vi "Visualizacion_NEW.vi"() -> ()   [LabVIEW 2021] (continued)
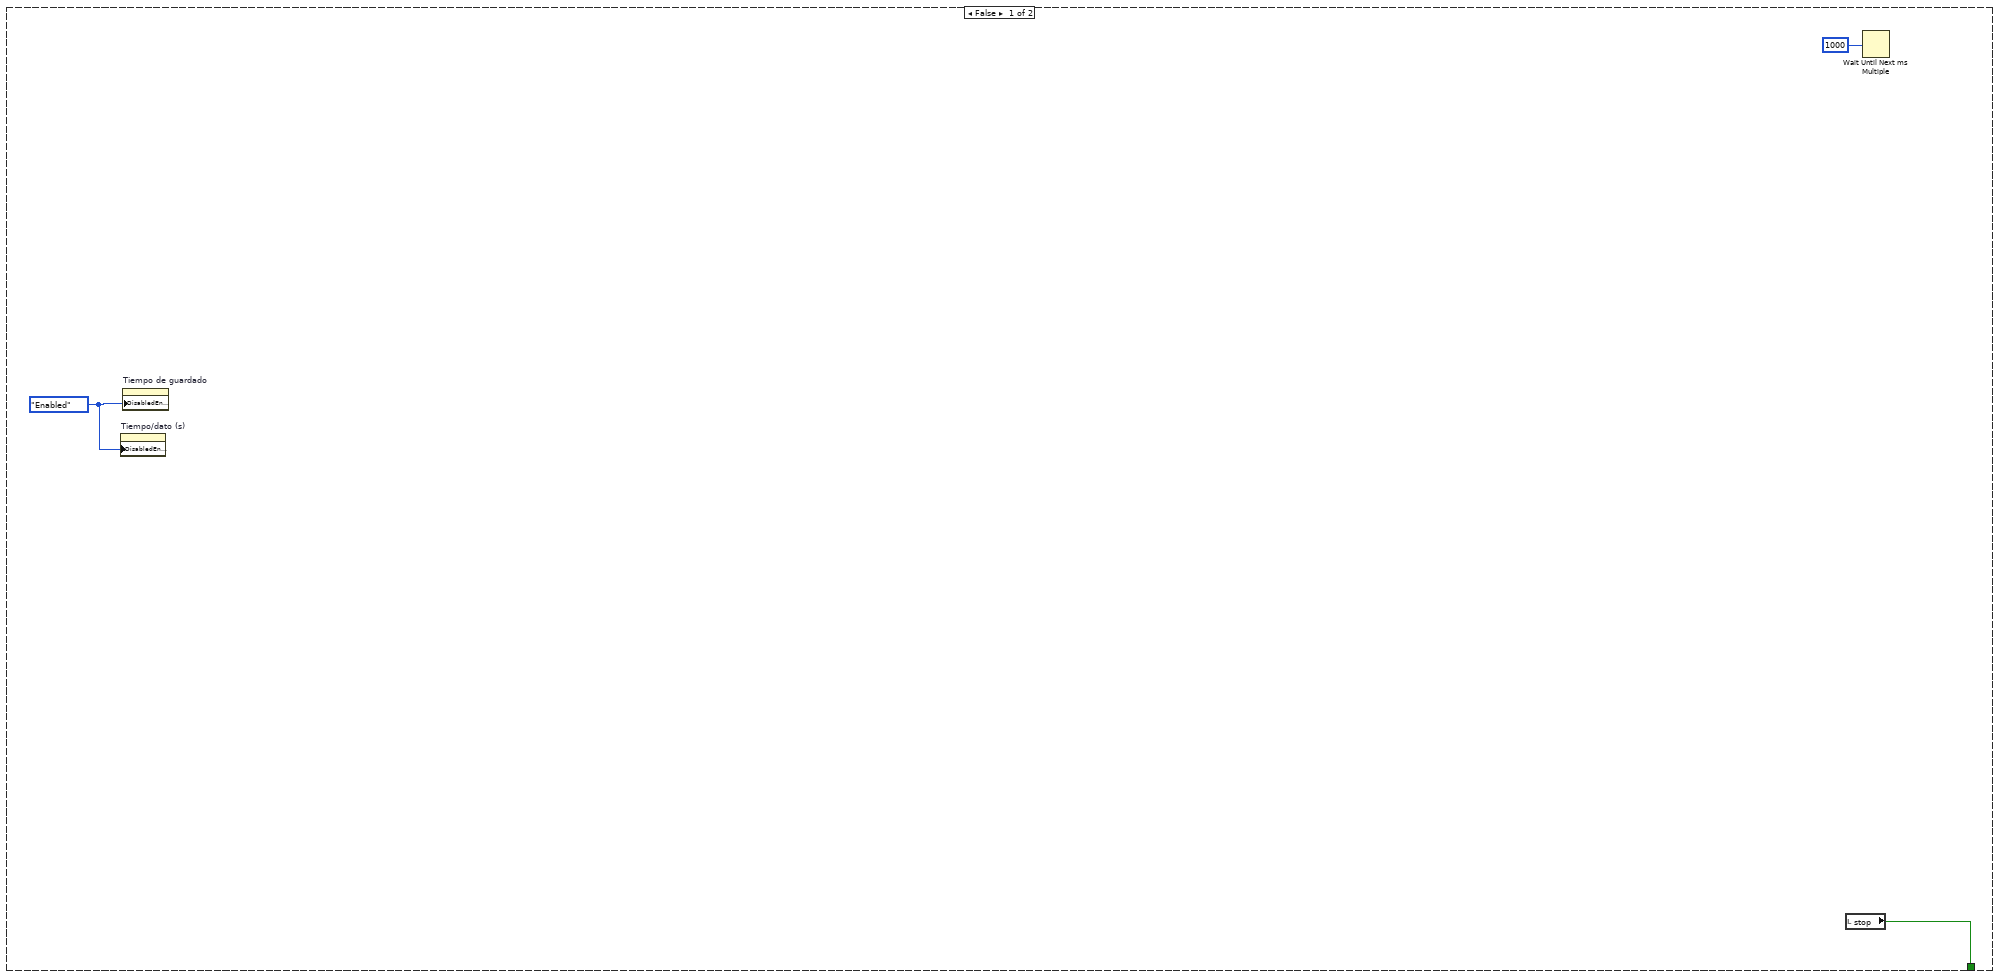
[diagram p2: hidden frame]
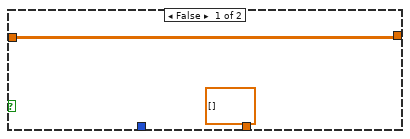
[diagram p3: hidden frame]
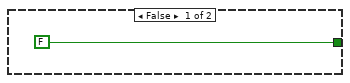
[diagram p4: hidden frame]
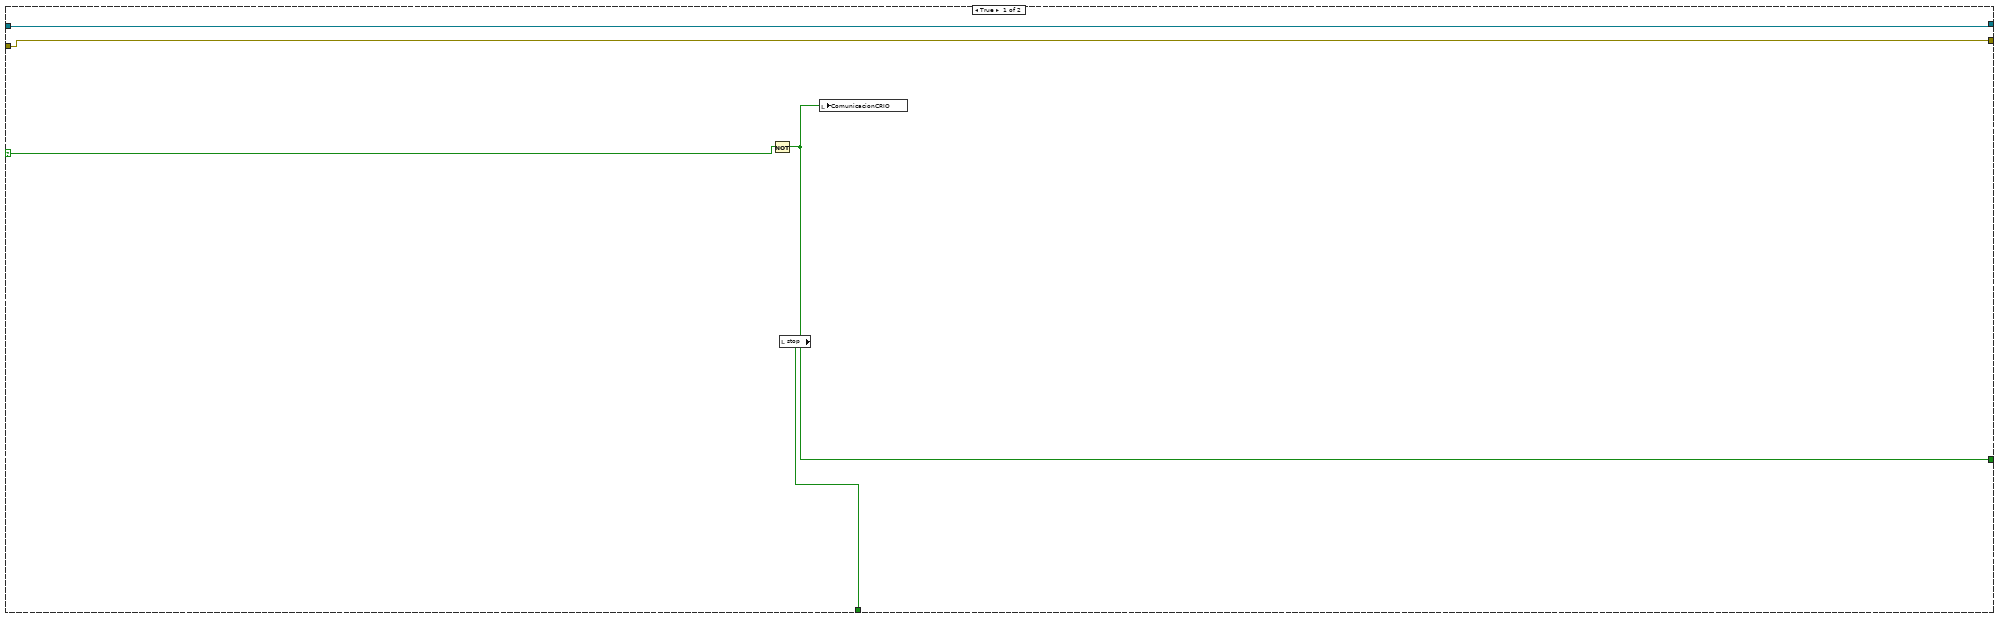
[diagram p6: hidden frame]
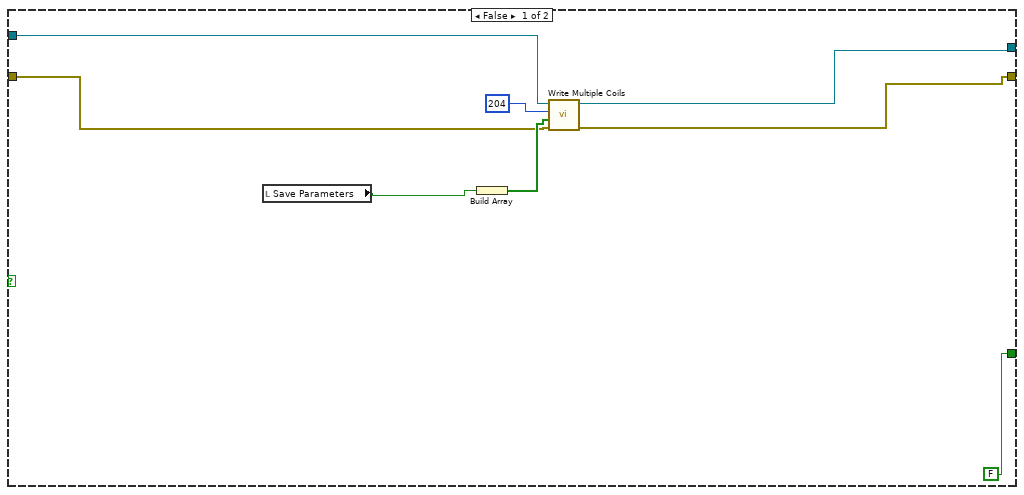
[diagram p8: hidden frame]
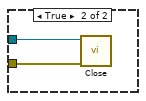
[diagram p9: hidden frame]
                frame False {
                }
                frame True {
                  n111 = flat-sequence {
                    tunnel: w160 -> [w172]
                    tunnel: w159 -> [w171]
                    tunnel: w158 -> [w170]
                    tunnel: w157 -> [w169]
                    tunnel: [w169] -> w155
                    tunnel: [w164] -> w152
                    tunnel: [w163] -> w150
                    tunnel: w155 -> [w185]
                    tunnel: [w185] -> w154
                    tunnel: [w184] -> w153
                    tunnel: w152 -> [w184]
                    tunnel: [w183] -> w151
                    tunnel: w150 -> [w183]
                    tunnel: [FALSE ("Warning saved")] -> w149
                    tunnel: [w189] -> w156
                    tunnel: w154 -> [w189]
                    tunnel: w153 -> [w188]
                    tunnel: w151 -> [w187]
                    tunnel: w149 -> [w186]
                    frame #0 {
                      n112 = disable-structure shown="Disabled" {
                        frame Disabled {
                          n113 = call <vilib>:"Application Directory.vi"() -> ("Application Directory"=w178:path)
                          n114 = Build Path(base path=w178) -> (appended path=w177:path)  [unwired: 1 in]
                          n115 = Build Path(base path=w177, name or relative path=path "data CC.tdms") -> ()  [unwired: 1 out]
                        }
                        frame Enabled {
                        }
                      }
                      n116 = TDMS Open(10:T6."open or create" ("operation (0:open)"), 11:w170) -> (0:w174:errorcluster, 3:w175:refnum<k34>)  [unwired: 5 in]
                      n117 = local read "W to save"() -> (w161:string[][])
                      n118 = TDMS Write(0:w175, 5:"Cámara climática" ("group name in (Untitled)"), 7:w172, 9:w171, 11:w174) -> (4:w168:refnum<k34>, 15:w167:errorcluster)  [unwired: 1 in, 2 out]
                      n119 = Transpose 2D Array(2D array=w161) -> (transposed array=w162:string[][])
                      n120 = TDMS Write(0:w168, 5:"Warnings y Errores" ("group name in (Untitled)"), 7:string[] ["Time", "id", "Description"] ("channel name(s) in (Untitled)"), 9:w162, 11:w167) -> (4:w163:refnum<k34>, 15:w164:errorcluster)  [unwired: 1 in, 2 out]
                    }
                    frame #1 {
                      n121 = local write "Warning saved"(TRUE ("Warning saved")) -> ()
                      n122 = Wait (ms)(milliseconds to wait=u32 300) -> ()  [unwired: 1 out]
                    }
                    frame #2 {
                      n123 = TDMS Close(8:w188, 11:w187) -> ()  [unwired: 2 out]
                      n124 = local write "Warning saved"(w186) -> ()
                    }
                  }
                }
              }
              n125 = Transpose 2D Array(2D array=w132) -> (transposed array=w131:dbl[][])
              n126 = Multiply(x="Tiempo/dato (s)", y=u32 1000) -> (x*y=w87:u32)
              n127 = Wait Until Next ms Multiple(millisecond multiple=w87) -> ()  [unwired: 1 out]
            }
          }
        }
      }
      n128 = while {
        tunnel: w18 -> [_]
        tunnel: w17 -> [_]
        tunnel: w16 -> [_]
        stop <- w190 stop-if-true
        n129 = flat-sequence {
          tunnel: [w199] -> w193
          tunnel: [w198] -> w192
          tunnel: [w197] -> w191
          tunnel: [w196] -> w190
          tunnel: w193 -> [w379]
          tunnel: w192 -> [w378]
          tunnel: w191 -> [w377]
          frame #0 {
            n130 = call-poly <vilib>:"Create Master Instance.vi"("address"="192.168.111.60") -> ("error out"=w195:errorcluster, "TCP master instance"=w200:refnum<class "Modbus Master.lvclass">)  [unwired: 9 in]
            "Comunicacion Modbus" <- w195
            n131 = Unbundle By Name(w195) -> ("status"=w194:bool)
            n132 = case shown="False" w194 {
              selector: w194 -> [w203 _]
              tunnel: w200 -> [w206 w212]
              tunnel: [w204 w211] -> w199
              tunnel: [w206 w210] -> w198
              tunnel: [w205 w209] -> w197
              tunnel: [w202 w208] -> w196
              tunnel: w195 -> [w205 w207]
              frame True {
                n133 = Not(x=w203) -> (.not. x?=w204:bool)
                n134 = local read "stop"() -> (w202:bool)
                n135 = local write "ComunicacionCRIO"(w204) -> ()
              }
              frame False {
                n136 = while {
                  shift-right: [w214] -> w210
                  shift-left: w212 -> [w282]
                  shift-right: [w213] -> w209
                  shift-left: w207 -> [w281]
                  tunnel: [w278] -> w211
                  tunnel: [w276] -> w208
                  stop <- w280 stop-if-true
                  n137 = call-dynamic "Read Coils.vi"("error in (no error)"=w281, "number of coils"=u16 23, "starting address"=u16 1, "Modbus master in"=w282) -> ("error out"=w267:errorcluster, "coil values"=w271:bool[], "Modbus master out"=w268:refnum<class "Modbus Master.lvclass">)  [unwired: 5 in]
                  n138 = local write "coil values"(w271) -> ()
                  n139 = call-dynamic "Read Coils.vi"("error in (no error)"=w267, "number of coils"=u16 1, "starting address"=u16 4, "Modbus master in"=w268) -> ("error out"=w265:errorcluster, "coil values"=w262:bool[], "Modbus master out"=w266:refnum<class "Modbus Master.lvclass">)  [unwired: 5 in]
                  n140 = Index Array(array=w262, index=0) -> (element=→"DO H2 Lab":bool)
                  n141 = call-dynamic "Read Holding Registers.vi"("error in (no error)"=w265, "number of holding registers"=u16 53, "starting address"=u16 100, "Modbus master in"=w266) -> ("error out"=w274:errorcluster, "register values"=w284:u16[], "Modbus master out"=w275:refnum<class "Modbus Master.lvclass">)  [unwired: 5 in]
                  n142 = Split 1D Array(array=w284, index=9) -> (first subarray=w283:u16[], second subarray=w288:u16[])
                  n143 = Array Size(array=w288) -> (size(s)=w287:i32)
                  n144 = Quotient & Remainder(x=w287, y=2) -> (floor(x/y)=w285:i32)  [unwired: 1 out]
                  n145 = for {
                    N: w285 -> [_]
                    tunnel: w288 -> [w369]
                    tunnel: [w366] -> w269 mode=indexing
                    i -> [w376]
                    n146 = Multiply(x=2, y=w376) -> (x*y=w374:i32)
                    n147 = Add(x=w374, y=1) -> (x+y=w372:i32)
                    n148 = Index Array(array=w369, index #1=w374, index #2=w372) -> (element #1=w371:u16, element #2=w370:u16)
                    n149 = Join Numbers(hi=w371, lo=w370) -> ((hi.lo)=w368:u32)
                    n150 = To Single Precision Float(number=w368) -> (single precision float=w365:sgl)
                    n151 = Subtract(x=w365, y=sgl 10000.0) -> (x-y=w363:sgl)
                    n152 = Divide(x=w363, y=sgl 100.0) -> (x/y=w366:sgl)
                  }
                  n153 = for {
                    tunnel: w283 -> [w362] mode=indexing
                    tunnel: [w360] -> w270 mode=indexing
                    n154 = Subtract(x=w362, y=u16 10000) -> (x-y=w360:u16)
                  }
                  n155 = local read "Coils write"() -> (w272:bool[])
                  n156 = local write "Int values"(w270) -> ()
                  n157 = local write "SGL values"(w269) -> ()
                  n158 = call-dynamic "Write Multiple Coils.vi"("error in (no error)"=w274, "coil values"=w272, "starting address"=u16 200, "Modbus master in"=w275) -> ("error out"=w255:errorcluster, "Modbus master out"=w256:refnum<class "Modbus Master.lvclass">)  [unwired: 6 in]
                  n159 = Build Array("Test PID (ºC)") -> (w253:bool[])
                  n160 = call-dynamic "Write Multiple Coils.vi"("error in (no error)"=w255, "coil values"=w253, "starting address"=u16 250, "Modbus master in"=w256) -> ("error out"=w229:errorcluster, "Modbus master out"=w230:refnum<class "Modbus Master.lvclass">)  [unwired: 6 in]
                  n161 = Build Array("Enable PI 1", "Enable PI 2", "Enable PI 3", "Enable PI 4", "Enable PI 5", "Enable PI 6", "Enable PI 7", "Enable PI 8") -> (w231:bool[])
                  n162 = call-dynamic "Write Multiple Coils.vi"("error in (no error)"=w229, "coil values"=w231, "starting address"=u16 240, "Modbus master in"=w230) -> ("error out"=w224:errorcluster, "Modbus master out"=w228:refnum<class "Modbus Master.lvclass">)  [unwired: 6 in]
                  n163 = Build Array("Descarte Media Temps") -> (w226:u16[])
                  n164 = Unbundle By Name(w255) -> ("status"=w279:bool)
                  n165 = call-dynamic "Write Multiple Holding Registers.vi"("error in (no error)"=w224, "holding register values"=w226, "starting address"=u16 350, "Modbus master in"=w228) -> ("error out"=w222:errorcluster, "Modbus master out"=w223:refnum<class "Modbus Master.lvclass">)  [unwired: 6 in]
                  n166 = local read "stop"() -> (w276:bool)
                  n167 = local read "Save Parameters"() -> (w259:bool)
                  n168 = Or(x=w279, y=w276) -> (x .or. y?=w280:bool)
                  n169 = Not(x=w279) -> (.not. x?=w278:bool)
                  "ComunicacionCRIO" <- w278
                  n170 = Build Array("TestPID 1(ºC)", "TestPID 2(ºC)", "TestPID3(ºC)", "TestPID 4(ºC)", "TestPID 5(ºC)", "TestPID 6(ºC)", "TestPID 7(ºC)", "TestPID 8(ºC)") -> (w250:u16[])
                  n171 = call-dynamic "Write Multiple Holding Registers.vi"("error in (no error)"=w222, "holding register values"=w250, "starting address"=u16 260, "Modbus master in"=w223) -> ("error out"=w257:errorcluster, "Modbus master out"=w258:refnum<class "Modbus Master.lvclass">)  [unwired: 6 in]
                  n172 = case shown="True" w259 {
                    tunnel: [FALSE ("Save Parameters") FALSE ("Save Parameters")] -> w241
                    tunnel: w258 -> [w313 w322]
                    tunnel: w257 -> [w312 w321]
                    tunnel: [w311 w320] -> w221
                    tunnel: [w310 w319] -> w220
                    frame False {
                      n173 = local read "Save Parameters"() -> (w314:bool)
                      n174 = Build Array(w314) -> (w316:bool[])
                      n175 = call-dynamic "Write Multiple Coils.vi"("error in (no error)"=w312, "coil values"=w316, "starting address"=u16 204, "Modbus master in"=w313) -> ("error out"=w310:errorcluster, "Modbus master out"=w311:refnum<class "Modbus Master.lvclass">)  [unwired: 6 in]
                    }
                    frame True {
                      n176 = for {
                        N: 3 -> [_]
                        shift-right: [w325] -> w320
                        shift-left: w322 -> [w327]
                        shift-right: [w324] -> w319
                        shift-left: w321 -> [w326]
                        n177 = Build Array("Save Parameters", "Digital Input Bitron Simulation") -> (w330:bool[])
                        n178 = call-dynamic "Write Multiple Coils.vi"("error in (no error)"=w326, "coil values"=w330, "starting address"=u16 204, "Modbus master in"=w327) -> ("error out"=w329:errorcluster, "Modbus master out"=w328:refnum<class "Modbus Master.lvclass">)  [unwired: 6 in]
                        n179 = Build Array("Setpoint corte frío(ºC)", "Setpoint Frío(ºC)", "Setpoint calor cam", "Setpoint calor corte rampa(ºC)", "Setpoint peltiers(ºC)", "Tiempo estabilidad de Frío(min)", "Tiempo mínimo de ciclo(min)", "Tiempo máximo de ciclo(min)", "Cam ºC/min", "Pelt ºC/min", "T ciclo (Bitron FSM Sim)") -> (w337:dbl[])
                        n180 = Array Size(array=w337) -> (size(s)=w336:i32)
                        n181 = for {
                          N: w336 -> [_]
                          shift-right: [w351] -> w334
                          shift-left: u16[] [0, 0, 0, 0, 0, 0, 0, 0, 0, 0, 0, 0, 0, 0, 0, 0, 0, 0, 0, 0, 0, 0] -> [w352]
                          tunnel: w337 -> [w350] mode=indexing
                          i -> [w359]
                          n182 = Multiply(x=2, y=w359) -> (x*y=w355:i32)
                          n183 = call "double_2u16.vi"("Entrada"=w350) -> ("Salida 2"=w356:u16, "Salida 1"=w357:u16)  [unwired: 9 in]
                          n184 = Add(x=1, y=w355) -> (x+y=w353:i32)
                          n185 = Replace Array Subset(array=w352, new element #1=w357, index #1=w355, new element #2=w356, index #2=w353) -> (w351:u16[])
                        }
                        n186 = call-dynamic "Write Multiple Holding Registers.vi"("error in (no error)"=w329, "holding register values"=w334, "starting address"=u16 300, "Modbus master in"=w328) -> ("error out"=w324:errorcluster, "Modbus master out"=w325:refnum<class "Modbus Master.lvclass">)  [unwired: 6 in]
                      }
                    }
                  }
                  n187 = local write "Save Parameters"(w241) -> ()
                  n188 = Wait (ms)(milliseconds to wait=u32 200) -> ()  [unwired: 1 out]
                  n189 = Build Array("Test PWM (%)") -> (w219:bool[])
                  n190 = call-dynamic "Write Multiple Coils.vi"("error in (no error)"=w220, "coil values"=w219, "starting address"=u16 400, "Modbus master in"=w221) -> ("error out"=w215:errorcluster, "Modbus master out"=w216:refnum<class "Modbus Master.lvclass">)  [unwired: 6 in]
                  n191 = case shown="True" "Test PWM (%)" {
                    tunnel: w216 -> [w295 w309]
                    tunnel: w215 -> [w294 w308]
                    tunnel: [w295 w307] -> w214
                    tunnel: [w294 w306] -> w213
                    frame False {
                    }
                    frame True {
                      n192 = Build Array("PWM 1(SP) 2", "PWM 2(SP) 2", "PWM 3(SP) 2", "PWM 4(SP)", "PWM 5(SP)", "PWM 6(SP)", "PWM 7(SP)", "PWM 8(SP)") -> (w296:u16[])
                      n193 = call-dynamic "Write Multiple Holding Registers.vi"("error in (no error)"=w308, "holding register values"=w296, "starting address"=u16 410, "Modbus master in"=w309) -> ("error out"=w306:errorcluster, "Modbus master out"=w307:refnum<class "Modbus Master.lvclass">)  [unwired: 6 in]
                    }
                  }
                }
              }
            }
          }
          frame #1 {
            n194 = case shown="False" w379 {
              tunnel: w378 -> [_ w381]
              tunnel: w377 -> [_ w380]
              frame False {
              }
              frame True {
                n195 = call-dynamic "Close.vi"("error in (no error)"=w380, "Modbus master in"=w381) -> ()  [unwired: 9 in, 1 out]
              }
            }
          }
          frame #2 {
            n196 = Tick Count (ms)() -> (millisecond timer value=w382:u32)
            n197 = while {
              tunnel: w382 -> [w388]
              stop <- w384 stop-if-true
              n198 = Tick Count (ms)() -> (millisecond timer value=w389:u32)
              n199 = local read "stop"() -> (w383:bool)
              n200 = Subtract(x=w389, y=w388) -> (x-y=w387:u32)
              n201 = Greater Or Equal?(x=w387, y=u32 5000) -> (x >= y?=w385:bool)
              n202 = Or(x=w385, y=w383) -> (x .or. y?=w384:bool)
            }
          }
        }
      }
      n203 = while {
        tunnel: w15 -> [_]
        stop <- "stop" stop-if-true
        # "MANIFOLD 8 Y BOBINA 8"
        # "manifold 7 y bobina 7"
        # "MANIFOLD 6 Y BOBINA 6"
        # "MANIFOLD 4 Y BOBINA 4"
        # "MANIFOLD Y BOBINA 3"
        # "MANIFOLD Y BOBINA 2"
        # "Manifold  y  Bobina 5"
        # "MANIFOLD 1 Y BOBINA 1"
        # "Visualizacion camara climatica"
        # "Control y visualizacion programa principal"
        n204 = local read "SGL values"() -> (w430:sgl[])
        n205 = local read "SGL values"() -> (w496:sgl[])
        n206 = local read "coil values"() -> (w490:bool[])
        n207 = local read "Temp Man 1"() -> (w474:sgl)
        n208 = local read "T bob 1"() -> (w473:dbl)
        n209 = local read "SP (T)"() -> (w475:sgl)
        n210 = Index Array(array=w430, index #18=21 ("index")) -> (element #1=→"SP (T)":sgl, element #2=→"Temp Man 1" →"T Man 1":sgl, element #3=→"Temp Man 2" →"T Man 2":sgl, element #4=→"Temp Man 3" →"T Man 3":sgl, element #5=→"Temp Man 4" →"T Man 4":sgl, element #6=→"Temp Man 5" →"T Man 5":sgl, element #7=→"Temp Man 6" →"T Man 6":sgl, element #8=→"Temp Man 7" →"T Man 7":sgl, element #9=→"Temp Man 8" →"T Man 8":sgl, element #10=→"Temp bob 1" →"T bob 1":sgl, element #11=→"Temp bob 2" →"T bob 2":sgl, element #12=→"Temp bob 3" →"T bob 3":sgl, element #13=→"Temp bob 4" →"T bob 4":sgl, element #14=→"Temp bob 5" →"T bob 5":sgl, element #15=→"Temp bob 6" →"T bob 6":sgl, element #16=→"Temp bob 7" →"T bob 7":sgl, element #17=→"Temp bob 8" →"T bob 8":sgl, element #18=w391:sgl)  [unwired: 17 in]
        "MEAN (T)" <- w391
        n211 = Index Array(array=w490, index=1) -> (element=→"Peltiers enable":bool)
        n212 = Index Array(array=w496, index #1=17 ("index")) -> (element #1=w494:sgl, element #2=w493:sgl, element #3=w492:sgl, element #4=w491:sgl)  [unwired: 3 in]
        "Humedad relativa (HR)" <- w494
        "Temperatura Camara" <- w492
        "Setpoint_hum_write" <- w493
        "Setpoint_temp_write" <- w491
        n213 = local read "MEAN (T)"() -> (w393:sgl)
        n214 = Merge Signals(w475, w474, w473) -> (→"VALVULA 1 Y BOBINA 1":dynamicdata)
        n215 = Get Date/Time In Seconds() -> (seconds since 1Jan1904=w498:timestamp)
        "current time" <- w498
        n216 = To Double Precision Float(number=w498) -> (double precision float=w392:dbl)
        n217 = Merge Signals(w494, w492, w493, w491, w393, w392) -> (→"Camara climatica":dynamicdata)
        n218 = local read "T Man 5"() -> (w459:dbl)
        n219 = local read "SP (T)"() -> (w460:sgl)
        n220 = local read "T bob 5"() -> (w458:dbl)
        n221 = local read "Int values"() -> (w472:u16[])
        n222 = Merge Signals(w460, w459, w458) -> (→"VALVULA 5  Y BOBINA 5":dynamicdata)
        n223 = local read "SP (T)"() -> (w433:sgl)
        n224 = local read "SP (T)"() -> (w454:sgl)
        n225 = local read "T Man 3"() -> (w453:dbl)
        n226 = local read "T bob 3"() -> (w452:dbl)
        n227 = Merge Signals(w433, w391) -> (→"TEMPERATURA MEDIA":dynamicdata)
        n228 = Index Array(array=w472) -> (element #1=→"Segmento_temp":u16, element #2=→"PWM 1(SP)":u16, element #3=→"PWM 2(SP)":u16, element #4=→"PWM 3(SP)":u16, element #5=→"PWM 4(SP)":u16, element #6=→"PWM 5(SP)":u16, element #7=→"PWM 6(SP)":u16, element #8=→"PWM 7(SP)":u16, element #9=→"PWM 8(SP)":u16)  [unwired: 9 in]
        n229 = Merge Signals(w454, w453, w452) -> (→"VALVULA 3 Y BOBINA 3":dynamicdata)
        n230 = local read "coil values"() -> (w480:bool[])
        n231 = local read "T Man 2"() -> (w447:dbl)
        n232 = local read "T bob 2"() -> (w446:dbl)
        n233 = local read "SP (T)"() -> (w456:sgl)
        n234 = local read "coil values"() -> (w487:bool[])
        n235 = Index Array(array=w480, index=2) -> (element=→"senal_bitron":bool)
        n236 = local read "coil values"() -> (w462:bool[])
        n237 = Index Array(array=w487, index=0) -> ()  [unwired: 1 out]
        n238 = Merge Signals(w456, w447, w446) -> (→"VALVULA 2 Y BOBINA 2":dynamicdata)
        n239 = local read "SP (T)"() -> (w450:sgl)
        n240 = local read "T Man 4"() -> (w449:dbl)
        n241 = local read "T bob 4"() -> (w448:dbl)
        n242 = Index Array(array=w462) -> (element #1=→"Program Status":bool)  [unwired: 9 in, 8 out]
        n243 = Merge Signals(w450, w449, w448) -> (→"VALVULA 4 Y BOBINA 4":dynamicdata)
        n244 = local read "SP (T)"() -> (w441:sgl)
        n245 = local read "T Man 7"() -> (w440:dbl)
        n246 = local read "T bob 7"() -> (w439:dbl)
        n247 = property on="PWM 1(SP)" class="DigNum (strict)" props=["Indicator"]() -> ()  [unwired: 2 in, 3 out]
        n248 = Merge Signals(w441, w440, w439) -> (→"VALVULA 7 Y BOBINA 7":dynamicdata)
        n249 = local read "SP (T)"() -> (w443:sgl)
        n250 = local read "T Man 6"() -> (w444:dbl)
        n251 = local read "T bob 6"() -> (w445:dbl)
        n252 = Build Array("run_program", "Pause", "Pause_Entrar_camara", "Stop Control Program") -> (→"Coils write":bool[])
        n253 = Merge Signals(w443, w444, w445) -> (→"VALVULA 6 Y BOBINA 6":dynamicdata)
        n254 = local read "Temp bob 8"() -> (w434:sgl)
        n255 = local read "T Man 8"() -> (w435:dbl)
        n256 = local read "SGL values"() -> (w412:sgl[])
        n257 = local read "SP (T)"() -> (w436:sgl)
        n258 = local read "MEAN (T)"() -> (w394:sgl)
        n259 = Merge Signals(w436, w435, w434) -> (→"VALVULA 8 Y PELTIER 8":dynamicdata)
        n260 = Index Array(array=w412) -> (element #1=w411:sgl, element #2=w410:sgl, element #3=w409:sgl, element #4=w408:sgl, element #5=w407:sgl, element #6=w406:sgl, element #7=w405:sgl, element #8=w404:sgl, element #9=w403:sgl, element #10=w402:sgl, element #11=w401:sgl, element #12=w400:sgl, element #13=w399:sgl, element #14=w398:sgl, element #15=w397:sgl, element #16=w396:sgl, element #17=w395:sgl)  [unwired: 17 in]
        n261 = Merge Signals(w411, w410, w409, w408, w407, w406, w405, w404, w403, w402, w401, w400, w399, w398, w397, w396, w395, w394) -> (→"ALL TOGETHER":dynamicdata)
        n262 = Wait (ms)(milliseconds to wait=u32 500) -> ()  [unwired: 1 out]
      }
      n263 = while {
        stop <- w36 stop-if-true
        n264 = local read "warnings table"() -> (w39:T3)
        n265 = local read "coil values"() -> (w65:bool[])
        n266 = Array Subset(array=w65, index=4, length=19) -> (w34:bool[])
        n267 = call "Historical Warnings (SubVI).vi"("Warnings bool array"=w34, "in"="Reset", "warnings table in"=w39) -> ("Warnings table out"=→"warnings table":T3)  [unwired: 8 in]
        n268 = Index Array(array=w65, index #1=20 ("index")) -> (element #1=→"W2":bool, element #2=→"W3":bool, element #3=→"W4":bool)  [unwired: 2 in]
        n269 = Array Subset(array=w65, index=4, length=16) -> (w48:bool[])
        n270 = Index Array(array=w48) -> (element #1=→"W1.1":bool, element #2=→"W1.2":bool, element #3=→"W1.3":bool, element #4=→"W1.4":bool, element #5=→"W1.5":bool, element #6=→"W1.6":bool, element #7=→"W1.7":bool, element #8=→"W1.8":bool, element #9=→"W1.9":bool, element #10=→"1.10":bool, element #11=→"W1.11":bool, element #12=→"W1.14":bool, element #13=→"W1.12":bool, element #14=→"W1.13":bool, element #15=→"W1.15":bool, element #16=→"W1.16":bool)  [unwired: 16 in]
        n271 = local read "stop"() -> (w36:bool)
        n272 = local read "W to save"() -> (w31:string[][])
        n273 = call "Saving_Warnings(SubVI).vi"("Warnings bool array"=w34, "Reset"="Warning saved", "W In"=w31) -> ("W Out"=→"W to save":string[][])  [unwired: 8 in]
        n274 = Wait (ms)(milliseconds to wait=u32 20) -> ()  [unwired: 1 out]
      }
    }
    frame #2 {
      n275 = local write "stop"(w501) -> ()
    }
  }
